vi "Dresden R2R Sputter 03.02.2018 IY24.vi"() -> ()   [LabVIEW 2009] (continued)
                                }
                                }
                                frame #3 {
                                n26178 = local read "Semi"() -> (w31407:bool)
                                n26179 = case shown="False" w31407 {
                                frame #0 {
                                n26180 = local read "Pc_bv_opened_ch2"() -> (w31408:bool)
                                n26181 = case shown="False" w31408 {
                                frame #0 {
                                n26182 = local write "Pc_bv2_auto_open"(TRUE ("Pc_bv1_auto_open")) -> ()
                                }
                                frame #1 {
                                }
                                }
                                }
                                frame #1 {
                                }
                                }
                                }
                                frame #4 {
                                n26183 = local read "Semi"() -> (w31410:bool)
                                n26184 = case shown="False" w31410 {
                                frame #0 {
                                n26185 = local read "Pc_bv_opened_ch2"() -> (w31411:bool)
                                n26186 = case shown="False" w31411 {
                                frame #0 {
                                n26187 = Wait (ms)(milliseconds to wait=u32 1000) -> ()  [unwired: 1 out]
                                }
                                frame #1 {
                                }
                                }
                                }
                                frame #1 {
                                }
                                }
                                }
                                frame #5 {
                                n26188 = local read "Semi"() -> (w31413:bool)
                                n26189 = case shown="False" w31413 {
                                frame #0 {
                                n26190 = while {
                                i -> [w31419]
                                stop <- w31415 stop-if-true
                                n26191 = local read "Pc_bv_opened_ch2"() -> (w31417:bool)
                                n26192 = Greater?(x=w31419, y=120) -> (0:w31418:bool)
                                n26193 = local read "Semi"() -> (w31416:bool)
                                n26194 = Compound Arithmetic op=OR(w31416, w31417, w31418) -> (w31415:bool)
                                n26195 = Wait (ms)(milliseconds to wait=u32 500) -> ()  [unwired: 1 out]
                                }
                                }
                                frame #1 {
                                }
                                }
                                }
                                frame #6 {
                                n26196 = local read "Semi"() -> (w31421:bool)
                                n26197 = case shown="False" w31421 {
                                frame #0 {
                                n26198 = local read "Pc_bv_opened_ch2"() -> (w31422:bool)
                                n26199 = case shown="False" w31422 {
                                frame #0 {
                                n26200 = local write "Error Message"("Start up process  cancelled\nbecause  PC-BV not opened.\nPlease check PC-BV1 connections." ("Error Message")) -> ()
                                n26201 = Wait (ms)(milliseconds to wait=u32 1000) -> ()  [unwired: 1 out]
                                }
                                frame #1 {
                                }
                                }
                                }
                                frame #1 {
                                }
                                }
                                }
                                }
                                }
                                frame #1 {
                                }
                                }
                                }
                                frame #1 {
                                n26202 = local read "Semi"() -> (w31425:bool)
                                n26203 = case shown="False" w31425 {
                                frame #0 {
                                n26204 = Wait (ms)(milliseconds to wait=u32 1000) -> ()  [unwired: 1 out]
                                n26205 = local write "SDC1 28"(TRUE ("SDC1 28")) -> ()
                                }
                                frame #1 {
                                }
                                }
                                }
                                }
                                }
                                frame #22 {
                                # "set ar zero"
                                n26206 = stacked-sequence {
                                frame #0 {
                                n26207 = local read "Semi"() -> (w31428:bool)
                                n26208 = case shown="False" w31428 {
                                frame #0 {
                                n26209 = stacked-sequence {
                                frame #0 {
                                n26210 = local read "Semi"() -> (w31429:bool)
                                n26211 = case shown="False" w31429 {
                                frame #0 {
                                n26212 = local write "Ar_auto_set_zero_ch2"(TRUE ("Ar_auto_set_zero_ch1")) -> ()
                                }
                                frame #1 {
                                }
                                }
                                }
                                frame #1 {
                                n26213 = local read "Semi"() -> (w31431:bool)
                                n26214 = case shown="False" w31431 {
                                frame #0 {
                                n26215 = while {
                                i -> [w31434]
                                stop <- w31433 stop-if-true
                                n26216 = Greater?(x=w31434, y=150) -> (0:w31433:bool)
                                n26217 = local read "Semi"() -> (w31432:bool)
                                n26218 = case shown="False" w31432 {
                                tunnel: [FALSE TRUE] -> _
                                frame #0 {
                                n26219 = Wait Until Next ms Multiple(millisecond multiple=u32 200) -> ()  [unwired: 1 out]
                                }
                                frame #1 {
                                }
                                }
                                }
                                }
                                frame #1 {
                                }
                                }
                                }
                                frame #2 {
                                n26220 = local read "Semi"() -> (w31439:bool)
                                n26221 = case shown="False" w31439 {
                                frame #0 {
                                n26222 = local read "Ar_sccm_act 6"() -> (w31441:dbl)
                                n26223 = Less?(x=w31441, y=1) -> (x < y?=w31440:bool)
                                n26224 = case shown="False" w31440 {
                                frame #0 {
                                n26225 = local write "Ar_auto_set_zero_ch2"(TRUE ("Ar_auto_set_zero_ch1")) -> ()
                                }
                                frame #1 {
                                }
                                }
                                }
                                frame #1 {
                                }
                                }
                                }
                                frame #3 {
                                n26226 = local read "Semi"() -> (w31444:bool)
                                n26227 = case shown="False" w31444 {
                                frame #0 {
                                n26228 = local read "Ar_sccm_act 6"() -> (w31446:dbl)
                                n26229 = Less?(x=w31446, y=1) -> (x < y?=w31445:bool)
                                n26230 = case shown="False" w31445 {
                                frame #0 {
                                n26231 = while {
                                i -> [w31452]
                                stop <- w31449 stop-if-true
                                n26232 = Greater?(x=w31452, y=150) -> (0:w31450:bool)
                                n26233 = local read "Semi"() -> (w31448:bool)
                                n26234 = case shown="True" w31448 {
                                tunnel: [FALSE FALSE] -> w31451
                                frame #0 {
                                }
                                frame #1 {
                                n26235 = Wait Until Next ms Multiple(millisecond multiple=u32 200) -> ()  [unwired: 1 out]
                                }
                                }
                                n26236 = Or(x=w31451, y=w31450) -> (x .or. y?=w31449:bool)
                                }
                                }
                                frame #1 {
                                }
                                }
                                }
                                frame #1 {
                                }
                                }
                                }
                                frame #4 {
                                n26237 = local read "Semi"() -> (w31457:bool)
                                n26238 = case shown="False" w31457 {
                                frame #0 {
                                n26239 = Wait (ms)(milliseconds to wait=u32 1000) -> ()  [unwired: 1 out]
                                }
                                frame #1 {
                                }
                                }
                                }
                                }
                                }
                                frame #1 {
                                }
                                }
                                }
                                frame #1 {
                                n26240 = local read "Semi"() -> (w31459:bool)
                                n26241 = case shown="False" w31459 {
                                frame #0 {
                                n26242 = local write "SDC1 26"(TRUE ("SDC1 26")) -> ()
                                n26243 = Wait (ms)(milliseconds to wait=u32 1000) -> ()  [unwired: 1 out]
                                }
                                frame #1 {
                                }
                                }
                                }
                                }
                                }
                                frame #23 {
                                # "sov-ar close"
                                n26244 = stacked-sequence {
                                frame #0 {
                                n26245 = local read "Semi"() -> (w31462:bool)
                                n26246 = case shown="False" w31462 {
                                frame #0 {
                                n26247 = while {
                                i -> [w31468]
                                stop <- w31463 stop-if-true
                                n26248 = Greater?(x=w31468, y=50) -> (0:w31467:bool)
                                n26249 = case shown="True" w31467 {
                                frame #0 {
                                }
                                frame #1 {
                                n26250 = local write "Semi"(TRUE ("Semi")) -> ()
                                n26251 = local write "Error Message"("Coating Process  \nwas cancelled.\nPlease check \nSOV-Ar connection." ("Error Message")) -> ()
                                }
                                }
                                n26252 = local read "Ch2_Sov_Ar_di"() -> (w31466:bool)
                                n26253 = case shown="True" w31466 {
                                tunnel: [TRUE FALSE] -> w31465
                                frame #0 {
                                }
                                frame #1 {
                                n26254 = local write "Ch2_Sov_Ar_do"(FALSE ("Ch1_WFC_do")) -> ()
                                n26255 = Wait Until Next ms Multiple(millisecond multiple=u32 200) -> ()  [unwired: 1 out]
                                }
                                }
                                n26256 = local read "Semi"() -> (w31464:bool)
                                n26257 = Or(x=w31465, y=w31464) -> (x .or. y?=w31463:bool)
                                }
                                }
                                frame #1 {
                                }
                                }
                                }
                                frame #1 {
                                n26258 = local read "Semi"() -> (w31476:bool)
                                n26259 = case shown="False" w31476 {
                                frame #0 {
                                n26260 = local write "SDC1 27"(TRUE ("SDC1 27")) -> ()
                                n26261 = Wait (ms)(milliseconds to wait=u32 1000) -> ()  [unwired: 1 out]
                                }
                                frame #1 {
                                }
                                }
                                }
                                }
                                }
                                frame #24 {
                                # "CC OPEN"
                                n26262 = stacked-sequence {
                                frame #0 {
                                n26263 = local read "Semi"() -> (w31479:bool)
                                n26264 = case shown="False" w31479 {
                                frame #0 {
                                n26265 = while {
                                i -> [w31485]
                                stop <- w31480 stop-if-true
                                n26266 = Greater?(x=w31485, y=50) -> (0:w31484:bool)
                                n26267 = case shown="True" w31484 {
                                frame #0 {
                                }
                                frame #1 {
                                n26268 = local write "Semi"(TRUE ("Semi")) -> ()
                                n26269 = local write "Error Message"("Coating Process  \nwas cancelled.\nPlease check \nBG-BV connection." ("Error Message")) -> ()
                                }
                                }
                                n26270 = local read "Ch2_Cc_on_off_di"() -> (w31483:bool)
                                n26271 = case shown="False" w31483 {
                                tunnel: [FALSE TRUE] -> w31482
                                frame #0 {
                                n26272 = local write "Ch2_Cc_on_off_do"(TRUE ("Ch1_WFC_do")) -> ()
                                n26273 = Wait Until Next ms Multiple(millisecond multiple=u32 200) -> ()  [unwired: 1 out]
                                }
                                frame #1 {
                                }
                                }
                                n26274 = local read "Semi"() -> (w31481:bool)
                                n26275 = Or(x=w31482, y=w31481) -> (x .or. y?=w31480:bool)
                                }
                                }
                                frame #1 {
                                }
                                }
                                }
                                frame #1 {
                                n26276 = local read "Semi"() -> (w31493:bool)
                                n26277 = case shown="False" w31493 {
                                frame #0 {
                                n26278 = while {
                                i -> [w31498]
                                stop <- w31496 stop-if-true
                                n26279 = Greater?(x=w31498, y=30) -> (0:w31494:bool)
                                n26280 = Wait Until Next ms Multiple(millisecond multiple=u32 1000) -> ()  [unwired: 1 out]
                                n26281 = local read "Semi"() -> (w31497:bool)
                                n26282 = Or(x=w31494, y=w31497) -> (x .or. y?=w31496:bool)
                                }
                                }
                                frame #1 {
                                }
                                }
                                }
                                frame #2 {
                                n26283 = local read "Semi"() -> (w31500:bool)
                                n26284 = case shown="False" w31500 {
                                frame #0 {
                                n26285 = local write "SDC1 27b"(TRUE ("SDC1 3")) -> ()
                                n26286 = Wait (ms)(milliseconds to wait=u32 1000) -> ()  [unwired: 1 out]
                                }
                                frame #1 {
                                }
                                }
                                }
                                }
                                }
                                frame #25 {
                                # "CHECK CHAMBER PRESSURE"
                                n26287 = stacked-sequence {
                                frame #0 {
                                n26288 = local read "Semi"() -> (w31503:bool)
                                n26289 = case shown="False" w31503 {
                                frame #0 {
                                n26290 = while {
                                i -> [w31511]
                                stop <- w31505 stop-if-true
                                n26291 = Greater?(x=w31511, y=300) -> (0:w31510:bool)
                                n26292 = case shown="True" w31510 {
                                frame #0 {
                                }
                                frame #1 {
                                n26293 = local write "Semi"(TRUE ("Semi")) -> ()
                                n26294 = local write "Error Message"("Coating Process cancelled.\nPlease check chamber \nconnections." ("Error Message")) -> ()
                                }
                                }
                                n26295 = local read "Ch_CC_press_ch2 2"() -> (w31504:dbl)
                                n26296 = Greater Or Equal?(x=w31504, y=5e-05 ("CHAMBER PRESSURE 6")) -> (x >= y?=w31508:bool)
                                n26297 = case shown="True" w31508 {
                                tunnel: [TRUE FALSE] -> w31507
                                frame #0 {
                                }
                                frame #1 {
                                n26298 = Wait Until Next ms Multiple(millisecond multiple=u32 200) -> ()  [unwired: 1 out]
                                }
                                }
                                n26299 = local read "Semi"() -> (w31506:bool)
                                n26300 = Or(x=w31507, y=w31506) -> (x .or. y?=w31505:bool)
                                }
                                }
                                frame #1 {
                                }
                                }
                                }
                                frame #1 {
                                n26301 = local read "Semi"() -> (w31518:bool)
                                n26302 = case shown="False" w31518 {
                                frame #0 {
                                n26303 = Wait (ms)(milliseconds to wait=u32 1000) -> ()  [unwired: 1 out]
                                n26304 = local write "SDC1 27c"(TRUE ("SDC1 10")) -> ()
                                }
                                frame #1 {
                                }
                                }
                                }
                                }
                                }
                                frame #26 {
                                # "encoder info  add to other web selection"
                                n26305 = stacked-sequence {
                                frame #0 {
                                n26306 = local read "Semi"() -> (w31521:bool)
                                n26307 = case shown="False" w31521 {
                                frame #0 {
                                n26308 = local read "R_Web_selection"() -> (w31522:enum32{"Web", "Other"})
                                n26309 = case shown="\"Web\", Default" w31522 {
                                frame #0 {
                                # "TC -ROLL"
                                n26310 = local read "Semi"() -> (w31523:bool)
                                n26311 = case shown="False" w31523 {
                                frame #0 {
                                n26312 = stacked-sequence {
                                frame #0 {
                                n26313 = local read "R Maximum diameter"() -> (w31524:dbl)
                                n26314 = local write "Change_Max Diameter"(w31524) -> ()
                                n26315 = Wait (ms)(milliseconds to wait=u32 300) -> ()  [unwired: 1 out]
                                }
                                frame #1 {
                                n26316 = local read "R Single DC Step1 Coating Power Active"() -> (w31526:bool)
                                n26317 = local read "R Single DC Step2 Coating Power Active"() -> (w31527:bool)
                                n26318 = local read "R Single DC Step3 Coating Power Active"() -> (w31528:bool)
                                n26319 = local read "R Single DC Step4 Coating Power Active"() -> (w31529:bool)
                                n26320 = local read "R Single DC Step5 Coating Power Active"() -> (w31530:bool)
                                n26321 = Boolean To (0,1)(Boolean=w31526) -> (0, 1=w31531:i16)
                                n26322 = Boolean To (0,1)(Boolean=w31527) -> (0, 1=w31532:i16)
                                n26323 = Boolean To (0,1)(Boolean=w31528) -> (0, 1=w31533:i16)
                                n26324 = Boolean To (0,1)(Boolean=w31529) -> (0, 1=w31534:i16)
                                n26325 = Boolean To (0,1)(Boolean=w31530) -> (0, 1=w31535:i16)
                                n26326 = Compound Arithmetic op=ADD(w31531, w31532, w31533, w31534, w31535) -> (w31537:i16)
                                n26327 = local read "R Single DC Interval length"() -> (w31536:dbl)
                                n26328 = Multiply(x=w31536, y=w31537) -> (x*y=w31538:dbl)
                                n26329 = local write "Total length"(w31538) -> ()
                                }
                                frame #2 {
                                n26330 = local write "Calculate 3"(TRUE ("Calculate_auto")) -> ()
                                }
                                frame #3 {
                                n26331 = Wait (ms)(milliseconds to wait=u32 1000) -> ()  [unwired: 1 out]
                                }
                                frame #4 {
                                n26332 = local read "Change_Max Diameter"() -> (w31542:dbl)
                                n26333 = Wait (ms)(milliseconds to wait=u32 200) -> ()  [unwired: 1 out]
                                n26334 = local write "Initial Min Diameter"(w31542) -> ()
                                }
                                frame #5 {
                                n26335 = local write "Calculate 2"(TRUE ("Calculate_auto")) -> ()
                                }
                                frame #6 {
                                n26336 = local write "Roll_side_select"(enum32{"Left to Right", "Right to Left"}."Right to Left" ("Roll_side_select")) -> ()
                                }
                                frame #7 {
                                n26337 = Wait (ms)(milliseconds to wait=u32 100) -> ()  [unwired: 1 out]
                                n26338 = local write "Parameters_auto_set"(TRUE ("Parameters_auto_set")) -> ()
                                }
                                frame #8 {
                                n26339 = while {
                                i -> [w31551]
                                stop <- w31547 stop-if-true
                                n26340 = Wait Until Next ms Multiple(millisecond multiple=u32 300) -> ()  [unwired: 1 out]
                                n26341 = Greater?(x=w31551, y=100) -> (0:w31548:bool)
                                n26342 = local read "Parameters_auto_set"() -> (w31552:bool)
                                n26343 = case shown="False" w31552 {
                                tunnel: [TRUE FALSE] -> w31549
                                frame #0 {
                                }
                                frame #1 {
                                }
                                }
                                n26344 = Or(x=w31549, y=w31548) -> (x .or. y?=w31547:bool)
                                }
                                }
                                frame #9 {
                                n26345 = local read "R Tension Value"() -> (w31556:dbl)
                                n26346 = Wait (ms)(milliseconds to wait=u32 200) -> ()  [unwired: 1 out]
                                n26347 = local write "TC2_set_value"(w31556) -> ()
                                }
                                frame #10 {
                                n26348 = local write "TC2_auto_set"(TRUE ("TC1_auto_set")) -> ()
                                }
                                frame #11 {
                                w31559 = u16 1 items=["1", "2", "3", "4"] ("Target Chamber Sensor")
                                n26349 = local write "Target Chamber Sensor"(w31559) -> ()
                                }
                                frame #12 {
                                n26350 = local read "Total length"() -> (w31560:dbl)
                                n26351 = local write "Region"(w31560) -> ()
                                }
                                frame #13 {
                                n26352 = local read "Semi"() -> (w31561:bool)
                                n26353 = case shown="False" w31561 {
                                frame #0 {
                                n26354 = local write "Start_roll"(TRUE ("Start_roll")) -> ()
                                n26355 = Wait (ms)(milliseconds to wait=u32 300) -> ()  [unwired: 1 out]
                                }
                                frame #1 {
                                }
                                }
                                }
                                frame #14 {
                                n26356 = local read "Semi"() -> (w31564:bool)
                                n26357 = case shown="False" w31564 {
                                frame #0 {
                                n26358 = while {
                                stop <- w31568 stop-if-true
                                n26359 = Wait Until Next ms Multiple(millisecond multiple=u32 200 ("milliseconds to wait")) -> ()  [unwired: 1 out]
                                n26360 = local read "Start_roll"() -> (w31566:bool)
                                n26361 = Not(x=w31566) -> (.not. x?=w31565:bool)
                                n26362 = local read "Semi"() -> (w31569:bool)
                                n26363 = Or(x=w31565, y=w31569) -> (x .or. y?=w31568:bool)
                                }
                                }
                                frame #1 {
                                }
                                }
                                }
                                }
                                }
                                frame #1 {
                                }
                                }
                                }
                                frame #1 {
                                n26364 = disable-structure shown="Disabled" {
                                frame #0 {
                                # "OTHER"
                                n26365 = local read "Semi"() -> (w31570:bool)
                                n26366 = case shown="False" w31570 {
                                frame #0 {
                                n26367 = stacked-sequence {
                                frame #0 {
                                n26368 = local read "Semi"() -> (w31571:bool)
                                n26369 = case shown="False" w31571 {
                                frame #0 {
                                n26370 = while {
                                i -> [w31577]
                                stop <- w31574 stop-if-true
                                n26371 = Greater?(x=w31577, y=50) -> (0:w31576:bool)
                                n26372 = case shown="True" w31576 {
                                frame #0 {
                                }
                                frame #1 {
                                n26373 = local write "Error Message"("" ("Error Message")) -> ()
                                n26374 = local write "Semi"(TRUE ("Semi")) -> ()
                                }
                                }
                                n26375 = local read "Casette_servo_start/stop_di"() -> (w31573:bool)
                                n26376 = case shown="False" w31573 {
                                tunnel: [FALSE TRUE] -> w31572
                                frame #0 {
                                n26377 = local write "Casette_servo_start/stop_do"(TRUE ("Casette_servo_left_direction_do")) -> ()
                                n26378 = Wait Until Next ms Multiple(millisecond multiple=u32 500) -> ()  [unwired: 1 out]
                                }
                                frame #1 {
                                }
                                }
                                n26379 = local read "Semi"() -> (w31575:bool)
                                n26380 = Or(x=w31572, y=w31575) -> (x .or. y?=w31574:bool)
                                }
                                }
                                frame #1 {
                                }
                                }
                                }
                                frame #1 {
                                n26381 = local read "Semi"() -> (w31585:bool)
                                n26382 = case shown="False" w31585 {
                                frame #0 {
                                n26383 = while {
                                i -> [w31591]
                                stop <- w31588 stop-if-true
                                n26384 = Greater?(x=w31591, y=50) -> (0:w31590:bool)
                                n26385 = case shown="True" w31590 {
                                frame #0 {
                                }
                                frame #1 {
                                n26386 = local write "Error Message"("" ("Error Message")) -> ()
                                n26387 = local write "Semi"(TRUE ("Semi")) -> ()
                                }
                                }
                                n26388 = local read "Casette_servo_left_direction_di"() -> (w31587:bool)
                                n26389 = case shown="False" w31587 {
                                tunnel: [FALSE TRUE] -> w31586
                                frame #0 {
                                n26390 = local write "Casette_servo_left_direction_do"(TRUE ("Casette_servo_left_direction_do")) -> ()
                                n26391 = Wait Until Next ms Multiple(millisecond multiple=u32 200) -> ()  [unwired: 1 out]
                                }
                                frame #1 {
                                }
                                }
                                n26392 = local read "Semi"() -> (w31589:bool)
                                n26393 = Or(x=w31586, y=w31589) -> (x .or. y?=w31588:bool)
                                }
                                }
                                frame #1 {
                                }
                                }
                                }
                                frame #2 {
                                # "casette motion"
                                n26394 = while {
                                i -> [w31601]
                                stop <- w31599 stop-if-true
                                n26395 = Greater?(x=w31601, y=200) -> (0:w31602:bool)
                                n26396 = case shown="True" w31602 {
                                frame #0 {
                                }
                                frame #1 {
                                n26397 = local write "Semi"(TRUE ("Semi")) -> ()
                                }
                                }
                                n26398 = local read "Counter_read_data"() -> (w31607:i16)
                                n26399 = Greater?(x=w31607, y=i16 0) -> (0:w31605:bool)
                                n26400 = case shown="True" w31605 {
                                tunnel: [TRUE TRUE] -> w31604
                                frame #0 {
                                }
                                frame #1 {
                                n26401 = local write "Casette_servo_start/stop_do"(FALSE ("Casette_servo_start/stop_do")) -> ()
                                n26402 = Wait Until Next ms Multiple(millisecond multiple=u32 200) -> ()  [unwired: 1 out]
                                }
                                }
                                n26403 = local read "Semi"() -> (w31603:bool)
                                n26404 = Or(x=w31604, y=w31603) -> (x .or. y?=w31599:bool)
                                }
                                }
                                frame #3 {
                                n26405 = local read "Semi"() -> (w31613:bool)
                                n26406 = case shown="False" w31613 {
                                frame #0 {
                                n26407 = while {
                                i -> [w31619]
                                stop <- w31616 stop-if-true
                                n26408 = Greater?(x=w31619, y=50) -> (0:w31618:bool)
                                n26409 = case shown="True" w31618 {
                                frame #0 {
                                }
                                frame #1 {
                                n26410 = local write "Error Message"("" ("Error Message")) -> ()
                                n26411 = local write "Semi"(TRUE ("Semi")) -> ()
                                }
                                }
                                n26412 = local read "Casette_servo_start/stop_di"() -> (w31615:bool)
                                n26413 = case shown="True" w31615 {
                                tunnel: [TRUE FALSE] -> w31614
                                frame #0 {
                                }
                                frame #1 {
                                n26414 = local write "Casette_servo_start/stop_do"(FALSE ("Casette_servo_left_direction_do")) -> ()
                                n26415 = Wait Until Next ms Multiple(millisecond multiple=u32 500) -> ()  [unwired: 1 out]
                                }
                                }
                                n26416 = local read "Semi"() -> (w31617:bool)
                                n26417 = Or(x=w31614, y=w31617) -> (x .or. y?=w31616:bool)
                                }
                                }
                                frame #1 {
                                }
                                }
                                }
                                frame #4 {
                                n26418 = local read "Semi"() -> (w31627:bool)
                                n26419 = case shown="False" w31627 {
                                frame #0 {
                                n26420 = Wait Until Next ms Multiple(millisecond multiple=u32 5000 ("millisecond multiple 3")) -> ()  [unwired: 1 out]
                                }
                                frame #1 {
                                }
                                }
                                }
                                frame #5 {
                                n26421 = local read "Semi"() -> (w31629:bool)
                                n26422 = case shown="False" w31629 {
                                frame #0 {
                                n26423 = while {
                                i -> [w31635]
                                stop <- w31632 stop-if-true
                                n26424 = Greater?(x=w31635, y=50) -> (0:w31634:bool)
                                n26425 = case shown="True" w31634 {
                                frame #0 {
                                }
                                frame #1 {
                                n26426 = local write "Error Message"("" ("Error Message")) -> ()
                                n26427 = local write "Semi"(TRUE ("Semi")) -> ()
                                }
                                }
                                n26428 = local read "Casette_servo_start/stop_di"() -> (w31631:bool)
                                n26429 = case shown="False" w31631 {
                                tunnel: [FALSE TRUE] -> w31630
                                frame #0 {
                                n26430 = local write "Casette_servo_start/stop_do"(TRUE ("Casette_servo_left_direction_do")) -> ()
                                n26431 = Wait Until Next ms Multiple(millisecond multiple=u32 500) -> ()  [unwired: 1 out]
                                }
                                frame #1 {
                                }
                                }
                                n26432 = local read "Semi"() -> (w31633:bool)
                                n26433 = Or(x=w31630, y=w31633) -> (x .or. y?=w31632:bool)
                                }
                                }
                                frame #1 {
                                }
                                }
                                }
                                frame #6 {
                                n26434 = local read "Semi"() -> (w31643:bool)
                                n26435 = case shown="False" w31643 {
                                frame #0 {
                                n26436 = while {
                                i -> [w31649]
                                stop <- w31646 stop-if-true
                                n26437 = Greater?(x=w31649, y=50) -> (0:w31648:bool)
                                n26438 = case shown="True" w31648 {
                                frame #0 {
                                }
                                frame #1 {
                                n26439 = local write "Error Message"("" ("Error Message")) -> ()
                                n26440 = local write "Semi"(TRUE ("Semi")) -> ()
                                }
                                }
                                n26441 = local read "Casette_servo_left_direction_di"() -> (w31645:bool)
                                n26442 = case shown="True" w31645 {
                                tunnel: [TRUE FALSE] -> w31644
                                frame #0 {
                                }
                                frame #1 {
                                n26443 = local write "Casette_servo_left_direction_do"(FALSE ("Casette_servo_left_direction_do")) -> ()
                                n26444 = Wait Until Next ms Multiple(millisecond multiple=u32 200) -> ()  [unwired: 1 out]
                                }
                                }
                                n26445 = local read "Semi"() -> (w31647:bool)
                                n26446 = Or(x=w31644, y=w31647) -> (x .or. y?=w31646:bool)
                                }
                                }
                                frame #1 {
                                }
                                }
                                }
                                frame #7 {
                                # "casette motion"
                                n26447 = while {
                                i -> [w31660]
                                stop <- w31657 stop-if-true
                                n26448 = Greater?(x=w31660, y=200) -> (0:w31661:bool)
                                n26449 = case shown="True" w31661 {
                                frame #0 {
                                }
                                frame #1 {
                                n26450 = local write "Semi"(TRUE ("Semi")) -> ()
                                }
                                }
                                n26451 = local read "Counter_read_data"() -> (w31665:i16)
                                n26452 = Less?(x=w31665, y=i16 0) -> (x < y?=w31664:bool)
                                n26453 = case shown="True" w31664 {
                                tunnel: [TRUE TRUE] -> w31663
                                frame #0 {
                                }
                                frame #1 {
                                n26454 = local write "Casette_servo_start/stop_do"(FALSE ("Casette_servo_start/stop_do")) -> ()
                                n26455 = Wait Until Next ms Multiple(millisecond multiple=u32 200) -> ()  [unwired: 1 out]
                                }
                                }
                                n26456 = local read "Semi"() -> (w31662:bool)
                                n26457 = Or(x=w31663, y=w31662) -> (x .or. y?=w31657:bool)
                                }
                                }
                                frame #8 {
                                n26458 = local read "Semi"() -> (w31671:bool)
                                n26459 = case shown="False" w31671 {
                                frame #0 {
                                n26460 = while {
                                i -> [w31677]
                                stop <- w31674 stop-if-true
                                n26461 = Greater?(x=w31677, y=50) -> (0:w31676:bool)
                                n26462 = case shown="True" w31676 {
                                frame #0 {
                                }
                                frame #1 {
                                n26463 = local write "Error Message"("" ("Error Message")) -> ()
                                n26464 = local write "Semi"(TRUE ("Semi")) -> ()
                                }
                                }
                                n26465 = local read "Casette_servo_start/stop_di"() -> (w31673:bool)
                                n26466 = case shown="True" w31673 {
                                tunnel: [TRUE FALSE] -> w31672
                                frame #0 {
                                }
                                frame #1 {
                                n26467 = local write "Casette_servo_start/stop_do"(FALSE ("Casette_servo_left_direction_do")) -> ()
                                n26468 = Wait Until Next ms Multiple(millisecond multiple=u32 500) -> ()  [unwired: 1 out]
                                }
                                }
                                n26469 = local read "Semi"() -> (w31675:bool)
                                n26470 = Or(x=w31672, y=w31675) -> (x .or. y?=w31674:bool)
                                }
                                }
                                frame #1 {
                                }
                                }
                                }
                                frame #9 {
                                n26471 = local read "Semi"() -> (w31685:bool)
                                n26472 = case shown="False" w31685 {
                                frame #0 {
                                }
                                frame #1 {